vi "USRP(receiver,4800).vi"() -> ()   [LabVIEW 2013]
uses:
  <vilib>/Analysis/2dsp.llb/Complex FFT.vi
  <vilib>/Analysis/2dsp.llb/Inverse Complex FFT.vi
  IS-95/receiver/4800/RAKE(4800).vi
  IS-95/receiver/4800/Combination device(4800).vi
  IS-95/receiver/common/path deletes.vi
  IS-95/receiver/common/Viterbi.vi
  IS-95/receiver/4800/FER(4800).vi
  IS-95/receiver/common/metrics.vi
  IS-95/transmitter/4800/syndrom(4800).vi
  <instrlib>/niUSRP/niUSRP Fetch Rx Data (CDB).vi
  <vilib>/ptbypt/Time Domain.llb/Peak Detector PtByPt.vi
  IS-95/receiver/4800/Gateway(4800).vi
  <vilib>/Analysis/NI_AALPro.lvlib
panel:
  in  "channel":i32=11
  in  "IQ rate":dbl=900000.0 format="%#_13g"
  in  "gain":dbl=21.0 format="%#_6f"
  in  "device name":refnum<k15>="192.168.10.2"
  in  "freq.":dbl=850000000.0 format="%#_6p"
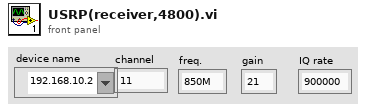
[diagram p1: front panel]
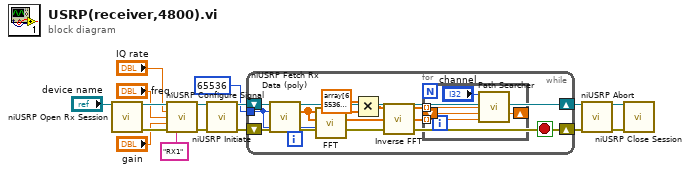
[diagram p0: block diagram]
diagram:
  n1 = call <instrlib>:"niUSRP Open Rx Session.vi"("device names"="device name") -> ("session handle out"=w16:refnum<k15>, "error out"=w15:errorcluster)  [unwired: 13 in]
  n2 = call <instrlib>:"niUSRP Configure Signal.vi"("session handle"=w16, "IQ rate"="IQ rate", "carrier frequency"="freq.", "gain"="gain", "error in (no error)"=w15, "active antenna"="RX1") -> ("session handle out"=w9:refnum<k15>, "error out"=w8:errorcluster)  [unwired: 5 in, 3 out]
  n3 = call <instrlib>:"niUSRP Initiate.vi"("session handle"=w9, "error in (no error)"=w8) -> ("session handle out"=w7:refnum<k15>, "error out"=w6:errorcluster)  [unwired: 12 in]
  n4 = while {
    shift-right: [w25] -> w4
    shift-left: w6 -> [w26]
    shift-right: [w22] -> w2
    shift-left: w7 -> [w23]
    tunnel: 65536 ("channel 2") -> [w18]
    stop <- w25 stop-if-true
    n5 = call-poly <instrlib>:"niUSRP Fetch Rx Data (poly).vi"("session handle"=w23, "number of samples"=w18, "error in (no error)"=w26) -> ("session handle out"=w22:refnum<k15>, "data"=w19:cdb[], "error out"=w25:errorcluster)  [unwired: 9 in, 1 out]
    n6 = call-poly <vilib>:"FFT.vi"("FFT size"=w18, "X"=w19) -> ("FFT {X}"=w21:cdb[])  [unwired: 8 in, 1 out]
    n7 = Multiply(x=cdb[] array[65536 elements] ("for path searcher"), y=w21) -> (x*y=w24:cdb[])
    n8 = call-poly <vilib>:"Inverse FFT.vi"("FFT {X}"=w24) -> ("X"=w20:cdb[])  [unwired: 9 in, 1 out]
    n9 = for {
      tunnel: w20 -> [w30] mode=indexing
      tunnel: w19 -> [w28] mode=indexing
      shift-right: [w28] -> _
      shift-left: _ -> [w27]
      n10 = call "Path Searcher.vi"("Номер\nканала"="channel", "corr"=w30, "sample"=w27) -> ()  [unwired: 13 in]
    }
  }
  n11 = call <instrlib>:"niUSRP Abort.vi"("session handle"=w2, "error in (no error)"=w4) -> ("session handle out"=w5:refnum<k15>, "error out"=w3:errorcluster)  [unwired: 12 in]
  n12 = call <instrlib>:"niUSRP Close Session.vi"("session handle"=w5, "error in (no error)"=w3) -> ()  [unwired: 13 in, 1 out]
